vi "UHR-Fleezers Control (host) - 10.2.vi"() -> ()   [LabVIEW 2009] (continued)
                        tunnel: w7403 -> [_ w7436]
                        tunnel: w7402 -> [_ w7427]
                        tunnel: w7392 -> [_ w7434]
                        tunnel: w7401 -> [_ w7433]
                        tunnel: w7390 -> [_ w7432]
                        tunnel: w7400 -> [_ w7431]
                        tunnel: w7385 -> [_ w7429]
                        tunnel: w7384 -> [_ w7428]
                        frame #0 {
                        }
                        frame #1 {
                          n1652 = local read "BD 1 Frequency 3 (MHz)"() -> (w7435:dbl)
                          n1653 = local read "BD 2 Frequency 3 (MHz)"() -> (w7430:dbl)
                          n1654 = local write "Trap Delta (MHz)"(w7427) -> ()
                          n1655 = property on="Initial delta (MHz)" class="DigNum (strict)"("Val(Sgnl)"=w7427) -> ()  [unwired: 2 in, 2 out]
                          n1656 = call "set RF board frequency - interlace.vi"("Board 2 Frequency Limits"=w7428, "Board 1 Frequency Limits"=w7429, "FPGA VI Reference In"=w7436, "Board 2 Frequency 3 (MHz)"=w7430, "Board 1 Frequency 3 (MHz)"=w7435, "Board 2 Frequency 2 (MHz)"=w7431, "Board 2 Frequency 1 (MHz)"=w7432, "Board 1 Frequency 2 (MHz)"=w7433, "Board 1 Frequency 1  (MHz)"=w7434) -> ()  [unwired: 1 in, 2 out]
                          n1657 = local write "BD 2 Frequency 1 (MHz)"(w7432) -> ()
                          n1658 = local write "BD 1 Frequency 1 (MHz)"(w7434) -> ()
                        }
                      }
                    }
                    frame #1 {
                    }
                  }
                }
                event #1 {
                  n1659 = event-data() -> ("Button"=w7437:u16)  [unwired: 8 out]
                  n1660 = case shown="3" w7437 {
                    tunnel: [FALSE TRUE] -> w7438
                    frame #0 {
                    }
                    frame #1 {
                      n1661 = local write "Manipulating Trap"(FALSE ("Manipulating Trap")) -> ()
                    }
                  }
                }
              }
            }
          }
        }
      }
      event #1 {
        n1662 = event-data() -> ()  [unwired: 6 out]
      }
    }
    n1663 = local read "Stop All"() -> (w7259:bool)
    n1664 = node-c288() -> ()  [unwired: 2 out]
  }
  n1665 = timed-loop "Run Scripts, including: stage motion" {
    tunnel: w42 -> [w7444]
    tunnel: w41 -> [w7445]
    tunnel: [w7445] -> w40
    tunnel: [w7444] -> w39
    timing: w37 -> [_]
    timing-out: [_] -> w36
    tunnel: w22 -> [w7443]
    tunnel: w23 -> [w7442]
    stop <- w7446 stop-if-true
    n1666 = node-c288() -> ()  [unwired: 1 in, 1 out]
    n1667 = event shown="[11] \"Take Force FB Data\nUpper Channel\": Value Change" {
      selector: _ -> [_ _ _ _ _ _ _ _ _ _ _ _ _ _ _ _ _]
      dyn-events: _ -> [_ _ _ _ _ _ _ _ _ _ _ _ _ _ _ _ _]
      timeout: _ -> [_ _ _ _ _ _ _ _ _ _ _ _ _ _ _ _ _]
      tunnel: ["Set Position" "Move to Position" "Move Cap. 1 (DNA Right)" "Move Cap. 2 (ADig Left)" _ "Cal/Data Acq. Spot" "Dump Beads" "Dip for Protein" _ _ "Got ADig bead" "Take Force FB Data\nUpper Channel" "Got DNA bead" "Take Stepping Data" _ "Take Detection Laser\nImage" _] -> _
      tunnel: [_ _ _ _ _ _ _ _ _ _ _ _ _ _ _ _ w7961] -> w7446
      tunnel: w7444 -> [w7464 w7472 w7496 w7551 w7596 w7632 w7710 w7735 w7785 w7811 _ w7840 _ _ _ _ _]
      tunnel: w7445 -> [w7465 w7473 w7497 w7552 w7597 w7633 w7711 w7736 w7786 w7812 _ w7841 _ _ _ _ _]
      tunnel: w7443 -> [_ _ w7494 w7548 _ _ _ _ _ _ _ _ _ _ _ _ _]
      tunnel: w7442 -> [_ _ w7493 w7549 _ _ _ _ _ _ _ _ _ _ _ _ _]
      event #0 {
        n1668 = event-data() -> ()  [unwired: 1 in, 5 out]
        n1669 = Build Array("Set Position 1", "Set Position 2", "Set Position 3", "Set Position 4", "Set Position 5") -> (w7463:bool[])
        n1670 = Boolean Array To Number(Boolean array=w7463) -> (number=w7462:u32)
        n1671 = Logarithm Base 2(1:w7462) -> (0:w7454:dbl)
        n1672 = call "Read Stage Position.vi"("error in"=w7464, "VISA resource name in"=w7465) -> ("Current Position"=w7469:cluster{dbl, dbl, dbl}, "error out"=w7468:errorcluster)  [unwired: 2 out]
        n1673 = Decrement(x="Position") -> (x-1=w7452:dbl)
        n1674 = Greater Or Equal?(x=w7454, y=0.0) -> (x >= y?=w7455:bool)
        n1675 = local write "Stage Control Serial Error"(w7468) -> ()
        n1676 = Cluster To Array(cluster=w7469) -> (array=w7466:dbl[])
        n1677 = Select(t=w7454, s=w7455, f=w7452) -> (s? t:f=w7451:dbl)
        n1678 = Increment(x=w7451) -> (x+1=w7450:dbl)
        n1679 = Build Array (concatenate)(w7450, w7466) -> (w7449:dbl[])
        n1680 = Replace Array Subset(array="Saved Stage Positions", new element=w7449, index (row)=w7451) -> (w7467:dbl[][])  [unwired: 1 in]
        n1681 = local write "Saved Stage Positions"(w7467) -> ()
      }
      event #1 {
        n1682 = event-data() -> ()  [unwired: 1 in, 5 out]
        n1683 = flat-sequence {
          tunnel: w7473 -> [w7476]
          tunnel: w7472 -> [w7475]
          frame #0 {
            n1684 = local read "Position"() -> (w7488:dbl)
            n1685 = local read "Saved Stage Positions"() -> (w7486:dbl[][])
            n1686 = Decrement(x=w7488) -> (x-1=w7485:dbl)
            n1687 = Array Subset(array=w7486, index (row)=w7485, length (row)=1 ("length"), index (col)=1 ("index"), length (col)=3 ("length")) -> (w7482:dbl[][])
            n1688 = Reshape Array(w7482, 3 ("dimension size")) -> (w7480:dbl[])
            n1689 = Array To Cluster(array=w7480) -> (cluster=w7479:cluster{"[0]":dbl, "[1]":dbl, "[2]":dbl})
            n1690 = call "Set Stage Position.vi"("Position"=w7479, "error in"=w7475, "VISA resource name in"=w7476) -> ("error out"=w7478:errorcluster)  [unwired: 2 out]
            n1691 = local write "Stage Control Serial Error"(w7478) -> ()
            n1692 = local write "Stage Moving"(TRUE ("Stage Moving")) -> ()
          }
          frame #1 {
            n1693 = call <vilib>:"Beep.vi"() -> ()  [unwired: 3 in, 9 out]
            n1694 = local write "Stage Moving"(FALSE ("Stage Moving")) -> ()
          }
        }
      }
      event #2 {
        n1695 = event-data() -> ()  [unwired: 1 in, 5 out]
        n1696 = local write "Move Cap. 1 (DNA Right)"(FALSE ("Move Cap. 1 (DNA Right)")) -> ()
        n1697 = flat-sequence {
          tunnel: w7497 -> [w7505]
          tunnel: w7496 -> [w7504]
          tunnel: w7494 -> [w7503]
          tunnel: w7493 -> [w7502]
          tunnel: [w7501] -> w7492
          tunnel: [w7500] -> w7491
          tunnel: ["Cap 1 Samp Flow ON"] -> w7490
          tunnel: w7492 -> [w7528]
          tunnel: w7491 -> [w7527]
          tunnel: w7490 -> [w7526]
          frame #0 {
            n1698 = local read "Saved Stage Positions"() -> (w7515:dbl[][])
            n1699 = Array Subset(array=w7515, index (row)=0 ("index"), length (row)=1 ("length"), index (col)=1 ("index"), length (col)=3 ("length")) -> (w7512:dbl[][])
            n1700 = Reshape Array(w7512, 3 ("dimension size")) -> (w7510:dbl[])
            n1701 = Array To Cluster(array=w7510) -> (cluster=w7509:cluster{"[0]":dbl, "[1]":dbl, "[2]":dbl})
            n1702 = case shown="True" "Cap 1 Samp Flow ON" {
              tunnel: w7502 -> [w7517 w7523]
              tunnel: w7503 -> [w7518 w7522]
              tunnel: [w7518 w7520] -> w7501
              tunnel: [w7517 w7519] -> w7500
              frame #0 {
              }
              frame #1 {
                # "run flow"
                n1703 = Concatenate Strings("run" ("string"), "\r") -> (w7524:string)
                n1704 = VISA Write(VISA resource name=w7522, write buffer=w7524, error in (no error)=w7523) -> (VISA resource name out=w7520:refnum<visa-resource-name>, error out=w7519:errorcluster)  [unwired: 1 out]
              }
            }
            n1705 = call "Set Stage Position.vi"("Position"=w7509, "error in"=w7504, "VISA resource name in"=w7505) -> ("error out"=w7508:errorcluster)  [unwired: 2 out]
            n1706 = local write "Stage Control Serial Error"(w7508) -> ()
            n1707 = local write "Stage Moving"(TRUE ("Stage Moving")) -> ()
          }
          frame #1 {
            n1708 = local write "Stage Moving"(FALSE ("Stage Moving")) -> ()
            n1709 = case shown="True" w7526 {
              tunnel: w7527 -> [w7533 w7539]
              tunnel: w7528 -> [w7534 w7538]
              tunnel: [w7534 w7536] -> _
              tunnel: [w7533 w7535] -> _
              frame #0 {
              }
              frame #1 {
                n1710 = Concatenate Strings("stop" ("string"), "\r") -> (w7540:string)
                n1711 = VISA Write(VISA resource name=w7538, write buffer=w7540, error in (no error)=w7539) -> (VISA resource name out=w7536:refnum<visa-resource-name>, error out=w7535:errorcluster)  [unwired: 1 out]
              }
            }
            n1712 = case shown="True" TRUE {
              tunnel: "Cap 1 T ON" -> [w7543 w7544]
              frame #0 {
                n1713 = property on="Trap 1 (ON/OFF)" class="Bool (strict)"("Val(Sgnl)"=w7543) -> ()  [unwired: 2 in, 2 out]
              }
              frame #1 {
                n1714 = property on="Trap 2 (ON/OFF)" class="Bool (strict)"("Val(Sgnl)"=w7544) -> ()  [unwired: 2 in, 2 out]
              }
            }
            n1715 = call <vilib>:"Beep.vi"() -> ()  [unwired: 3 in, 9 out]
            n1716 = case shown="True" "Cap 1 Flow ON" {
              frame #0 {
              }
              frame #1 {
                n1717 = property on="Inject Pump 1" class="Bool (strict)"("Val(Sgnl)"=TRUE ("Value (Signaling)")) -> ()  [unwired: 2 in, 2 out]
              }
            }
          }
        }
      }
      event #3 {
        n1718 = event-data() -> ()  [unwired: 1 in, 5 out]
        n1719 = local write "Move Cap. 2 (ADig Left)"(FALSE ("Move Cap. 2 (ADig Left)")) -> ()
        n1720 = flat-sequence {
          tunnel: w7552 -> [w7560]
          tunnel: w7551 -> [w7559]
          tunnel: w7549 -> [w7558]
          tunnel: w7548 -> [w7557]
          tunnel: [w7556] -> w7547
          tunnel: [w7555] -> w7546
          tunnel: ["Cap 2 Samp Flow ON"] -> w7545
          tunnel: w7547 -> [w7583]
          tunnel: w7546 -> [w7582]
          tunnel: w7545 -> [w7581]
          frame #0 {
            n1721 = local read "Saved Stage Positions"() -> (w7570:dbl[][])
            n1722 = case shown="True" "Cap 2 Samp Flow ON" {
              tunnel: w7558 -> [w7572 w7578]
              tunnel: w7557 -> [w7573 w7577]
              tunnel: [w7573 w7575] -> w7556
              tunnel: [w7572 w7574] -> w7555
              frame #0 {
              }
              frame #1 {
                # "run flow"
                n1723 = Concatenate Strings("run" ("string"), "\r") -> (w7579:string)
                n1724 = VISA Write(VISA resource name=w7577, write buffer=w7579, error in (no error)=w7578) -> (VISA resource name out=w7575:refnum<visa-resource-name>, error out=w7574:errorcluster)  [unwired: 1 out]
              }
            }
            n1725 = Array Subset(array=w7570, index (row)=1 ("index"), length (row)=1 ("length"), index (col)=1 ("index"), length (col)=3 ("length")) -> (w7567:dbl[][])
            n1726 = Reshape Array(w7567, 3 ("dimension size")) -> (w7565:dbl[])
            n1727 = Array To Cluster(array=w7565) -> (cluster=w7564:cluster{"[0]":dbl, "[1]":dbl, "[2]":dbl})
            n1728 = call "Set Stage Position.vi"("Position"=w7564, "error in"=w7559, "VISA resource name in"=w7560) -> ("error out"=w7563:errorcluster)  [unwired: 2 out]
            n1729 = local write "Stage Moving"(TRUE ("Stage Moving")) -> ()
            n1730 = local write "Stage Control Serial Error"(w7563) -> ()
          }
          frame #1 {
            n1731 = local write "Stage Moving"(FALSE ("Stage Moving")) -> ()
            n1732 = case shown="True" TRUE {
              tunnel: "Cap 2 T ON" -> [w7594 w7595]
              frame #0 {
                n1733 = property on="Trap 2 (ON/OFF)" class="Bool (strict)"("Val(Sgnl)"=w7594) -> ()  [unwired: 2 in, 2 out]
              }
              frame #1 {
                n1734 = property on="Trap 1 (ON/OFF)" class="Bool (strict)"("Val(Sgnl)"=w7595) -> ()  [unwired: 2 in, 2 out]
              }
            }
            n1735 = call <vilib>:"Beep.vi"() -> ()  [unwired: 3 in, 9 out]
            n1736 = case shown="True" w7581 {
              tunnel: w7583 -> [_ w7589]
              tunnel: w7582 -> [_ w7588]
              frame #0 {
              }
              frame #1 {
                n1737 = Concatenate Strings("stop" ("string"), "\r") -> (w7591:string)
                n1738 = VISA Write(VISA resource name=w7589, write buffer=w7591, error in (no error)=w7588) -> ()  [unwired: 3 out]
              }
            }
            n1739 = case shown="True" "Cap 2 Flow ON" {
              frame #0 {
              }
              frame #1 {
                n1740 = property on="Inject Pump 3" class="Bool (strict)"("Val(Sgnl)"=TRUE ("Value (Signaling)")) -> ()  [unwired: 2 in, 2 out]
              }
            }
          }
        }
      }
      event #4 {
        n1741 = event-data() -> ()  [unwired: 1 in, 5 out]
        n1742 = flat-sequence {
          tunnel: w7596 -> [w7618]
          tunnel: w7597 -> [w7598]
          frame #0 {
            n1743 = call "Read Stage Position.vi"("error in"=w7618, "VISA resource name in"=w7598) -> ("Current Position"=w7603:cluster{dbl, dbl, dbl}, "error out"=w7616:errorcluster, "VISA resource name out"=w7617:refnum<visa-resource-name>)  [unwired: 1 out]
            n1744 = local read "Saved Stage Positions"() -> (w7627:dbl[][])
            n1745 = Divide(x="z nudge increment (um)", y=1000.0) -> (x/y=w7615:dbl)
            n1746 = Boolean To (0,1)(Boolean="+z") -> (0, 1=w7607:i16)
            n1747 = Boolean To (0,1)(Boolean="-z") -> (0, 1=w7608:i16)
            n1748 = Array Subset(array=w7627, index (row)=1 ("index"), length (row)=1 ("length"), index (col)=1 ("index"), length (col)=3 ("length")) -> (w7624:dbl[][])
            n1749 = Multiply(x=w7607, y=w7615) -> (x*y=w7611:dbl)
            n1750 = Multiply(x=w7608, y=w7615) -> (x*y=w7609:dbl)
            n1751 = Unbundle(w7603) -> (w7601:dbl, w7600:dbl, w7604:dbl)
            n1752 = Negate(x=w7609) -> (-x=w7610:dbl)
            n1753 = Reshape Array(w7624, 3 ("dimension size")) -> (w7622:dbl[])
            n1754 = Add(x=w7611, y=w7610) -> (x+y=w7612:dbl)
            n1755 = Array To Cluster(array=w7622) -> ()  [unwired: 1 out]
            n1756 = Add(x=w7612, y=w7604) -> (x+y=w7602:dbl)
            n1757 = Bundle(cluster=w7603, w7601, w7600, w7602) -> (w7599:cluster{dbl, dbl, dbl})
            n1758 = call "Set Stage Position.vi"("Position"=w7599, "error in"=w7616, "VISA resource name in"=w7617) -> ("error out"=w7621:errorcluster)  [unwired: 2 out]
            n1759 = local write "Stage Moving"(TRUE ("Stage Moving")) -> ()
            n1760 = local write "Stage Control Serial Error"(w7621) -> ()
          }
          frame #1 {
            n1761 = local write "Stage Moving"(FALSE ("Stage Moving")) -> ()
            n1762 = call <vilib>:"Beep.vi"() -> ()  [unwired: 3 in, 9 out]
          }
        }
      }
      event #5 {
        n1763 = event-data() -> ()  [unwired: 1 in, 5 out]
        n1764 = flat-sequence {
          tunnel: w7633 -> [w7636]
          tunnel: w7632 -> [w7635]
          tunnel: ["Cal @ (MHz)"] -> w7630
          tunnel: w7630 -> [w7656]
          tunnel: w7630 -> [w7677]
          frame #0 {
            n1765 = local read "Saved Stage Positions"() -> (w7639:dbl[][])
            n1766 = Array Subset(array=w7639, index (row)=2 ("index"), length (row)=1 ("length"), index (col)=1 ("index"), length (col)=3 ("length")) -> (w7642:dbl[][])
            n1767 = Reshape Array(w7642, 3 ("dimension size")) -> (w7644:dbl[])
            n1768 = local write "Stage Moving"(TRUE ("Stage Moving")) -> ()
            n1769 = Array To Cluster(array=w7644) -> (cluster=w7645:cluster{"[0]":dbl, "[1]":dbl, "[2]":dbl})
            n1770 = call "Set Stage Position.vi"("Position"=w7645, "error in"=w7635, "VISA resource name in"=w7636) -> ("error out"=w7646:errorcluster)  [unwired: 2 out]
            n1771 = local write "Stage Control Serial Error"(w7646) -> ()
          }
          frame #1 {
            n1772 = property on="Trap Delta (MHz)" class="DigNum (strict)"("Val(Sgnl)"="Cal @ (MHz)") -> ()  [unwired: 2 in, 2 out]
            n1773 = local write "Stage Moving"(FALSE ("Stage Moving")) -> ()
            n1774 = call <vilib>:"Beep.vi"() -> ()  [unwired: 3 in, 9 out]
          }
          frame #2 {
            n1775 = Wait (ms)(milliseconds to wait=u32 100) -> ()  [unwired: 1 out]
          }
          frame #3 {
            n1776 = property on="Save Calibration" class="Bool (strict)"("Val(Sgnl)"=TRUE ("Value (Signaling)")) -> ()  [unwired: 2 in, 2 out]
          }
          frame #4 {
            n1777 = Wait (ms)(milliseconds to wait=u32 4000) -> ()  [unwired: 1 out]
          }
          frame #5 {
            n1778 = while {
              stop <- w7653 stop-if-true
              n1779 = local read "Saving..."() -> (w7654:bool)
              n1780 = Wait (ms)(milliseconds to wait=u32 100) -> ()  [unwired: 1 out]
              n1781 = Not(x=w7654) -> (.not. x?=w7653:bool)
            }
          }
          frame #6 {
            n1782 = case shown="True" "W/ Offset 1" {
              tunnel: w7656 -> [_ w7658]
              frame #0 {
              }
              frame #1 {
                n1783 = stacked-sequence {
                  tunnel: w7658 -> [_ _ _ _ _ _ _ w7675]
                  frame #0 {
                    n1784 = property on="Trap Delta (MHz)" class="DigNum (strict)"("Val(Sgnl)"="Offset 1 Start (MHz)") -> ()  [unwired: 2 in, 2 out]
                    n1785 = Replace Array Subset(array=u32[] [0] ("Index Values"), new element="Offset 1 Set", index=0) -> (w7659:u32[])
                    n1786 = property on="Saved AOD Raster Scan Parameter Sets" class="Arr (strict)"("Index Values"=w7659) -> ()  [unwired: 2 in, 2 out]
                  }
                  frame #1 {
                    n1787 = Wait (ms)(milliseconds to wait=u32 200) -> ()  [unwired: 1 out]
                  }
                  frame #2 {
                    n1788 = property on="Load parameters" class="Bool (strict)"("Val(Sgnl)"=TRUE ("Value (Signaling)")) -> ()  [unwired: 2 in, 2 out]
                  }
                  frame #3 {
                    n1789 = Wait (ms)(milliseconds to wait=u32 200) -> ()  [unwired: 1 out]
                  }
                  frame #4 {
                    n1790 = property on="Trap Raster Scan" class="Bool (strict)"("Val(Sgnl)"=TRUE ("Value (Signaling)")) -> ()  [unwired: 2 in, 2 out]
                  }
                  frame #5 {
                    n1791 = Wait (ms)(milliseconds to wait=u32 2000) -> ()  [unwired: 1 out]
                  }
                  frame #6 {
                    n1792 = while {
                      stop <- w7672 stop-if-true
                      n1793 = local read "Raster Scanning..."() -> (w7674:bool)
                      n1794 = local read "Saving..."() -> (w7670:bool)
                      n1795 = Wait (ms)(milliseconds to wait=u32 100) -> ()  [unwired: 1 out]
                      n1796 = Not(x=w7670) -> (.not. x?=w7669:bool)
                      n1797 = Not(x=w7674) -> (.not. x?=w7671:bool)
                      n1798 = And(x=w7671, y=w7669) -> (x .and. y?=w7672:bool)
                    }
                  }
                  frame #7 {
                    n1799 = property on="Trap Delta (MHz)" class="DigNum (strict)"("Val(Sgnl)"=w7675) -> ()  [unwired: 2 in, 2 out]
                  }
                }
              }
            }
          }
          frame #7 {
            n1800 = local read "Save ave N"() -> (w7676:dbl)
            n1801 = case shown="True" "W/ Offset 2" {
              tunnel: w7677 -> [_ w7683]
              tunnel: w7676 -> [_ w7682]
              frame #0 {
                n1802 = Multiply(x="Cal read wait (s)", y=u32 1000 ("milliseconds to wait")) -> (x*y=w7680:u32)
                n1803 = Wait (ms)(milliseconds to wait=w7680) -> ()  [unwired: 1 out]
              }
              frame #1 {
                n1804 = stacked-sequence {
                  tunnel: w7683 -> [_ _ _ _ _ _ _ _ _ w7704 _ _]
                  tunnel: w7682 -> [_ _ _ _ _ _ _ _ _ w7702 _ _]
                  frame #0 {
                    n1805 = property on="Save ave N" class="DigNum (strict)"("Val(Sgnl)"=1.0 ("Value (Signaling)")) -> ()  [unwired: 2 in, 2 out]
                  }
                  frame #1 {
                    n1806 = Wait (ms)(milliseconds to wait=u32 500) -> ()  [unwired: 1 out]
                  }
                  frame #2 {
                    n1807 = property on="Trap Delta (MHz)" class="DigNum (strict)"("Val(Sgnl)"="Offset 2 Start (MHz)") -> ()  [unwired: 2 in, 2 out]
                    n1808 = Replace Array Subset(array=u32[] [0] ("Index Values"), new element="Offset 2 Set", index=0) -> (w7688:u32[])
                    n1809 = property on="Saved AOD Raster Scan Parameter Sets" class="Arr (strict)"("Index Values"=w7688) -> ()  [unwired: 2 in, 2 out]
                  }
                  frame #3 {
                    n1810 = Wait (ms)(milliseconds to wait=u32 500) -> ()  [unwired: 1 out]
                  }
                  frame #4 {
                    n1811 = property on="Load parameters" class="Bool (strict)"("Val(Sgnl)"=TRUE ("Value (Signaling)")) -> ()  [unwired: 2 in, 2 out]
                  }
                  frame #5 {
                    n1812 = Wait (ms)(milliseconds to wait=u32 500) -> ()  [unwired: 1 out]
                  }
                  frame #6 {
                    n1813 = property on="Trap Raster Scan" class="Bool (strict)"("Val(Sgnl)"=TRUE ("Value (Signaling)")) -> ()  [unwired: 2 in, 2 out]
                  }
                  frame #7 {
                    n1814 = Wait (ms)(milliseconds to wait=u32 2000) -> ()  [unwired: 1 out]
                  }
                  frame #8 {
                    n1815 = while {
                      stop <- w7697 stop-if-true
                      n1816 = local read "Raster Scanning..."() -> (w7700:bool)
                      n1817 = local read "Saving..."() -> (w7698:bool)
                      n1818 = Wait (ms)(milliseconds to wait=u32 100) -> ()  [unwired: 1 out]
                      n1819 = Not(x=w7698) -> (.not. x?=w7696:bool)
                      n1820 = Not(x=w7700) -> (.not. x?=w7699:bool)
                      n1821 = And(x=w7699, y=w7696) -> (x .and. y?=w7697:bool)
                    }
                  }
                  frame #9 {
                    n1822 = property on="Trap Delta (MHz)" class="DigNum (strict)"("Val(Sgnl)"=w7704) -> ()  [unwired: 2 in, 2 out]
                    n1823 = property on="Saved AOD Raster Scan Parameter Sets" class="Arr (strict)"("Index Values"=u32[] [0]) -> ()  [unwired: 2 in, 2 out]
                    n1824 = property on="Save ave N" class="DigNum (strict)"("Val(Sgnl)"=w7702) -> ()  [unwired: 2 in, 2 out]
                  }
                  frame #10 {
                    n1825 = Wait (ms)(milliseconds to wait=u32 500) -> ()  [unwired: 1 out]
                  }
                  frame #11 {
                    n1826 = property on="Load parameters" class="Bool (strict)"("Val(Sgnl)"=TRUE ("Value (Signaling)")) -> ()  [unwired: 2 in, 2 out]
                  }
                }
              }
            }
          }
          frame #8 {
            n1827 = property on="Read Cal" class="Bool (strict)"("Val(Sgnl)"=TRUE ("Value (Signaling)")) -> ()  [unwired: 2 in, 2 out]
          }
          frame #9 {
            n1828 = Wait (ms)(milliseconds to wait=u32 500) -> ()  [unwired: 1 out]
          }
          frame #10 {
            n1829 = property on="Fish for Tether" class="Bool (strict)"("Val(Sgnl)"=TRUE ("Value (Signaling)")) -> ()  [unwired: 2 in, 2 out]
          }
        }
        n1830 = local write "Cal/Data Acq. Spot"(FALSE ("Cal/Data Acq. Spot")) -> ()
      }
      event #6 {
        n1831 = event-data() -> ()  [unwired: 1 in, 5 out]
        n1832 = flat-sequence {
          tunnel: w7711 -> [w7717]
          tunnel: w7710 -> [w7716]
          frame #0 {
            w7713 = FALSE ("Fl. Triggered...")
            w7714 = TRUE ("Stage Moving")
            n1833 = local read "Saving..."() -> (w7715:bool)
            n1834 = local write "Fl. Triggered..."(w7713) -> ()
            n1835 = local write "Stage Moving"(w7714) -> ()
            n1836 = property on="Green Laser ON/Interlacing" class="Bool (strict)"("Val(Sgnl)"=w7713) -> ()  [unwired: 2 in, 2 out]
            n1837 = property on="Trap Pos. FB ON" class="Bool (strict)"("Val(Sgnl)"=w7713) -> ()  [unwired: 2 in, 2 out]
            n1838 = local write "Tether"(w7713) -> ()
            n1839 = local write "Stop Saving"(w7715) -> ()
            n1840 = property on="Sample Channel Flow" class="Bool (strict)"("Val(Sgnl)"=w7714) -> ()  [unwired: 2 in, 2 out]
          }
          frame #1 {
            n1841 = local read "Saved Stage Positions"() -> (w7718:dbl[][])
            n1842 = Array Subset(array=w7718, index (row)=3 ("index"), length (row)=1 ("length"), index (col)=1 ("index"), length (col)=3 ("length")) -> (w7723:dbl[][])
            n1843 = Reshape Array(w7723, 3 ("dimension size")) -> (w7721:dbl[])
            n1844 = Array To Cluster(array=w7721) -> (cluster=w7720:cluster{"[0]":dbl, "[1]":dbl, "[2]":dbl})
            n1845 = call "Set Stage Position.vi"("Position"=w7720, "error in"=w7716, "VISA resource name in"=w7717) -> ()  [unwired: 3 out]
          }
          frame #2 {
            w7727 = FALSE ("Value (Signaling)")
            n1846 = property on="Trap 1 (ON/OFF)" class="Bool (strict)"("Val(Sgnl)"=w7727) -> ()  [unwired: 2 in, 2 out]
            n1847 = property on="Trap 2 (ON/OFF)" class="Bool (strict)"("Val(Sgnl)"=w7727) -> ()  [unwired: 2 in, 2 out]
            n1848 = call <vilib>:"Beep.vi"() -> ()  [unwired: 3 in, 9 out]
          }
          frame #3 {
            n1849 = property on="Move Cap. 2 (ADig Left)" class="Bool (strict)"("Val(Sgnl)"=TRUE ("Value (Signaling)")) -> ()  [unwired: 2 in, 2 out]
          }
        }
      }
      event #7 {
        n1850 = event-data() -> ()  [unwired: 1 in, 5 out]
        n1851 = flat-sequence {
          tunnel: w7735 -> [w7739]
          tunnel: w7736 -> [w7740]
          tunnel: [w7740] -> w7730
          tunnel: [w7739] -> w7729
          tunnel: [w7743] -> w7733
          tunnel: [w7742] -> w7731
          tunnel: w7730 -> [w7746]
          tunnel: w7729 -> [w7745]
          tunnel: [w7756] -> w7734
          tunnel: w7733 -> [w7756]
          tunnel: [w7755] -> w7732
          tunnel: w7731 -> [w7755]
          tunnel: w7734 -> [w7761]
          tunnel: w7732 -> [w7760]
          frame #0 {
            n1852 = case shown="True" "Move Trap Before?" {
              frame #0 {
              }
              frame #1 {
                n1853 = property on="Trap Delta (MHz)" class="DigNum (strict)"("Val(Sgnl)"="Dip Trap Delta 1 (MHz)") -> ()  [unwired: 2 in, 2 out]
              }
            }
          }
          frame #1 {
            n1854 = local read "Saved Stage Positions"() -> (w7744:dbl[][])
            n1855 = Array Subset(array=w7744, index (row)=4 ("index"), length (row)=1 ("length"), index (col)=1 ("index"), length (col)=3 ("length")) -> (w7751:dbl[][])
            n1856 = Reshape Array(w7751, 3 ("dimension size")) -> (w7749:dbl[])
            n1857 = Array To Cluster(array=w7749) -> (cluster=w7748:cluster{"[0]":dbl, "[1]":dbl, "[2]":dbl})
            n1858 = call "Set Stage Position.vi"("Position"=w7748, "error in"=w7745, "VISA resource name in"=w7746) -> ("error out"=w7742:errorcluster, "VISA resource name out"=w7743:refnum<visa-resource-name>)  [unwired: 1 out]
          }
          frame #2 {
            n1859 = Multiply(x="Duration (s)", y=1000.0) -> (x*y=w7757:dbl)
            n1860 = Wait (ms)(milliseconds to wait=w7757) -> ()  [unwired: 1 out]
          }
          frame #3 {
            n1861 = local read "Saved Stage Positions"() -> (w7762:dbl[][])
            n1862 = Array Subset(array=w7762, index (row)=2 ("index"), length (row)=1 ("length"), index (col)=1 ("index"), length (col)=3 ("length")) -> (w7767:dbl[][])
            n1863 = Reshape Array(w7767, 3 ("dimension size")) -> (w7765:dbl[])
            n1864 = Array To Cluster(array=w7765) -> (cluster=w7764:cluster{"[0]":dbl, "[1]":dbl, "[2]":dbl})
            n1865 = call "Set Stage Position.vi"("Position"=w7764, "error in"=w7760, "VISA resource name in"=w7761) -> ()  [unwired: 3 out]
          }
          frame #4 {
            n1866 = case shown="True" "Move Trap After?" {
              frame #0 {
              }
              frame #1 {
                n1867 = property on="Trap Delta (MHz)" class="DigNum (strict)"("Val(Sgnl)"="Dip Trap Delta 2 (MHz)") -> ()  [unwired: 2 in, 2 out]
              }
            }
          }
          frame #5 {
            n1868 = case shown="True" "Green ON After?" {
              frame #0 {
              }
              frame #1 {
                n1869 = property on="Green Laser ON/Interlacing" class="Bool (strict)"("Val(Sgnl)"=TRUE ("Value (Signaling)")) -> ()  [unwired: 2 in, 2 out]
              }
            }
          }
          frame #6 {
            n1870 = Wait (ms)(milliseconds to wait=u32 500) -> ()  [unwired: 1 out]
          }
          frame #7 {
            n1871 = case shown="True" "Save Data After?" {
              frame #0 {
              }
              frame #1 {
                n1872 = property on="Start Saving" class="Bool (strict)"("Val(Sgnl)"=TRUE ("Value (Signaling)")) -> ()  [unwired: 2 in, 2 out]
              }
            }
          }
        }
      }
      event #8 {
        n1873 = event-data() -> ()  [unwired: 1 in, 5 out]
        n1874 = flat-sequence {
          tunnel: w7786 -> [w7789]
          tunnel: w7785 -> [w7797]
          tunnel: [w7791] -> w7784
          tunnel: [w7790] -> w7783
          tunnel: [w7788] -> w7781
          tunnel: [w7787] -> w7778
          tunnel: w7784 -> [w7804]
          tunnel: w7783 -> [w7803]
          tunnel: [w7801] -> w7782
          tunnel: w7781 -> [w7802]
          tunnel: [w7800] -> w7780
          tunnel: [w7799] -> w7779
          tunnel: w7778 -> [w7799]
          tunnel: w7782 -> [w7808]
          tunnel: w7780 -> [w7807]
          tunnel: w7779 -> [w7806]
          frame #0 {
            n1875 = call "Read Stage Position.vi"("error in"=w7797, "VISA resource name in"=w7789) -> ("Current Position"=w7787:cluster{dbl, dbl, dbl}, "error out"=w7790:errorcluster, "VISA resource name out"=w7788:refnum<visa-resource-name>)  [unwired: 1 out]
            "Current Position" <- w7787
            n1876 = local write "Stage Control Serial Error"(w7790) -> ()
            n1877 = Unbundle(w7787) -> (w7794:dbl, w7796:dbl, w7792:dbl)
            n1878 = Add(x=w7796, y="Y change (mm)") -> (x+y=w7793:dbl)
            n1879 = Bundle(w7794, w7793, w7792) -> (w7791:cluster{dbl, dbl, dbl})  [unwired: 1 in]
          }
          frame #1 {
            # "move to new position and start saving"
            n1880 = local write "Stage Moving"(TRUE ("Stage Moving")) -> ()
            n1881 = local write "Start Saving"(TRUE ("Start Saving")) -> ()
            n1882 = call "Set Stage Position.vi"("Position"=w7804, "error in"=w7803, "VISA resource name in"=w7802) -> ("error out"=w7800:errorcluster, "VISA resource name out"=w7801:refnum<visa-resource-name>)  [unwired: 1 out]
          }
          frame #2 {
            # "go back to start"
            n1883 = call "Set Stage Position.vi"("Position"=w7806, "error in"=w7807, "VISA resource name in"=w7808) -> ()  [unwired: 3 out]
          }
          frame #3 {
            # "stop saving"
            n1884 = local write "Stop Saving"(TRUE ("Stop Saving")) -> ()
            n1885 = local write "Stage Moving"(FALSE ("Stage Moving")) -> ()
          }
        }
      }
      event #9 {
        n1886 = event-data() -> ()  [unwired: 1 in, 5 out]
        n1887 = Or(x="Move to Position 5", y="Lower Ch. Cap.") -> (x .or. y?=w7814:bool)
        n1888 = Build Array("Move to Position 1", "Move to Position 2", "Move to Position 3", "Move to Position 4", w7814) -> (w7817:bool[])
        n1889 = Boolean Array To Number(Boolean array=w7817) -> (number=w7816:u32)
        n1890 = Logarithm Base 2(1:w7816) -> (0:w7815:dbl)
        n1891 = flat-sequence {
          tunnel: w7815 -> [w7826]
          tunnel: w7812 -> [w7824]
          tunnel: w7811 -> [w7823]
          frame #0 {
            n1892 = local read "Saved Stage Positions"() -> (w7834:dbl[][])
            n1893 = Array Subset(array=w7834, index (row)=w7826, length (row)=1 ("length"), index (col)=1 ("index"), length (col)=3 ("length")) -> (w7831:dbl[][])
            n1894 = Reshape Array(w7831, 3 ("dimension size")) -> (w7829:dbl[])
            n1895 = Array To Cluster(array=w7829) -> (cluster=w7828:cluster{"[0]":dbl, "[1]":dbl, "[2]":dbl})
            n1896 = call "Set Stage Position.vi"("Position"=w7828, "error in"=w7823, "VISA resource name in"=w7824) -> ("error out"=w7827:errorcluster)  [unwired: 2 out]
            n1897 = local write "Stage Moving"(TRUE ("Stage Moving")) -> ()
            n1898 = local write "Stage Control Serial Error"(w7827) -> ()
          }
          frame #1 {
            n1899 = call <vilib>:"Beep.vi"() -> ()  [unwired: 3 in, 9 out]
            n1900 = local write "Stage Moving"(FALSE ("Stage Moving")) -> ()
          }
        }
      }
      event #10 {
        n1901 = event-data() -> ()  [unwired: 1 in, 5 out]
        n1902 = property on="Move Cap. 1 (DNA Right)" class="Bool (strict)"("Val(Sgnl)"=TRUE ("Value (Signaling)")) -> ()  [unwired: 2 in, 2 out]
        n1903 = property on="Inject Pump 3" class="Bool (strict)"("Val(Sgnl)"=FALSE ("Value (Signaling)")) -> ()  [unwired: 2 in, 2 out]
      }
      event #11 {
        n1904 = event-data() -> ()  [unwired: 1 in, 5 out]
        n1905 = flat-sequence {
          tunnel: w7841 -> [w7845]
          tunnel: w7840 -> [w7844]
          frame #0 {
            n1906 = local read "Saved Stage Positions"() -> (w7848:dbl[][])
            n1907 = local write "Stage Moving"(TRUE ("Stage Moving")) -> ()
            n1908 = Array Subset(array=w7848, index (row)=4 ("index"), length (row)=1 ("length"), index (col)=1 ("index"), length (col)=3 ("length")) -> (w7853:dbl[][])
            n1909 = Reshape Array(w7853, 3 ("dimension size")) -> (w7851:dbl[])
            n1910 = Array To Cluster(array=w7851) -> (cluster=w7846:cluster{"[0]":dbl, "[1]":dbl, "[2]":dbl})
            n1911 = call "Set Stage Position.vi"("Position"=w7846, "error in"=w7844, "VISA resource name in"=w7845) -> ("error out"=w7843:errorcluster)  [unwired: 2 out]
            n1912 = local write "Stage Control Serial Error"(w7843) -> ()
          }
          frame #1 {
            n1913 = call <vilib>:"Beep.vi"() -> ()  [unwired: 3 in, 9 out]
            n1914 = property on="Trap Delta (MHz)" class="DigNum (strict)"("Val(Sgnl)"="Starting \nTrap Delta (MHz)") -> ()  [unwired: 2 in, 2 out]
            n1915 = local write "Stage Moving"(FALSE ("Stage Moving")) -> ()
            n1916 = Wait (ms)(milliseconds to wait=u32 1000) -> ()  [unwired: 1 out]
          }
          frame #2 {
            n1917 = property on="Set SP to Reading" class="Bool (strict)"("Val(Sgnl)"=TRUE ("Value (Signaling)")) -> ()  [unwired: 2 in, 2 out]
            n1918 = Wait (ms)(milliseconds to wait=u32 500) -> ()  [unwired: 1 out]
          }
          frame #3 {
            w7862 = TRUE ("Value (Signaling)")
            n1919 = property on="Trap Pos. FB ON" class="Bool (strict)"("Val(Sgnl)"=w7862) -> ()  [unwired: 2 in, 2 out]
            n1920 = property on="Green Laser ON/Interlacing" class="Bool (strict)"("Val(Sgnl)"=w7862) -> ()  [unwired: 2 in, 2 out]
            n1921 = Wait (ms)(milliseconds to wait=u32 500) -> ()  [unwired: 1 out]
          }
          frame #4 {
            n1922 = property on="Start Saving" class="Bool (strict)"("Val(Sgnl)"=TRUE ("Value (Signaling)")) -> ()  [unwired: 2 in, 2 out]
          }
        }
      }
      event #12 {
        n1923 = event-data() -> ()  [unwired: 1 in, 5 out]
        n1924 = property on="Cal/Data Acq. Spot" class="Bool (strict)"("Val(Sgnl)"=TRUE ("Value (Signaling)")) -> ()  [unwired: 2 in, 2 out]
        n1925 = property on="Inject Pump 1" class="Bool (strict)"("Val(Sgnl)"=FALSE ("Value (Signaling)")) -> ()  [unwired: 2 in, 2 out]
      }
      event #13 {
        n1926 = event-data() -> ()  [unwired: 1 in, 5 out]
        n1927 = local read "Save ave N"() -> (w7875:dbl)
        n1928 = flat-sequence {
          tunnel: w7875 -> [w7877]
          tunnel: [w7877] -> w7870
          tunnel: [w7879] -> w7871
          tunnel: w7870 -> [w7879]
          tunnel: [w7881] -> w7872
          tunnel: w7871 -> [w7881]
          tunnel: [w7884] -> w7873
          tunnel: w7872 -> [w7884]
          tunnel: [w7886] -> w7874
          tunnel: w7873 -> [w7886]
          tunnel: [w7888] -> w7868
          tunnel: w7874 -> [w7888]
          tunnel: w7868 -> [w7891]
          tunnel: [w7891] -> w7867
          tunnel: w7867 -> [w7892]
          tunnel: [w7892] -> w7869
          tunnel: w7869 -> [w7898]
          frame #0 {
            n1929 = property on="Save ave N" class="DigNum (strict)"("Val(Sgnl)"="Save ave factor") -> ()  [unwired: 2 in, 2 out]
          }
          frame #1 {
            n1930 = Wait (ms)(milliseconds to wait=u32 100) -> ()  [unwired: 1 out]
          }
          frame #2 {
            n1931 = local read "Offset 2 Start (MHz)"() -> (w7883:dbl)
            n1932 = property on="Saved AOD Raster Scan Parameter Sets" class="Arr (strict)"("Index Values"=u32[] [2]) -> ()  [unwired: 2 in, 2 out]
            n1933 = property on="Trap Delta (MHz)" class="DigNum (strict)"("Val(Sgnl)"=w7883) -> ()  [unwired: 2 in, 2 out]
          }
          frame #3 {
            n1934 = property on="Load parameters" class="Bool (strict)"("Val(Sgnl)"=TRUE ("Value (Signaling)")) -> ()  [unwired: 2 in, 2 out]
          }
          frame #4 {
            n1935 = Wait (ms)(milliseconds to wait=u32 100) -> ()  [unwired: 1 out]
          }
          frame #5 {
            n1936 = property on="Trap Raster Scan" class="Bool (strict)"("Val(Sgnl)"=TRUE ("Value (Signaling)")) -> ()  [unwired: 2 in, 2 out]
          }
          frame #6 {
            n1937 = Wait (ms)(milliseconds to wait=u32 1000) -> ()  [unwired: 1 out]
          }
          frame #7 {
            n1938 = while {
              stop <- w7895 stop-if-true
              n1939 = local read "Raster Scanning..."() -> (w7897:bool)
              n1940 = local read "Saving..."() -> (w7896:bool)
              n1941 = Not(x=w7896) -> (.not. x?=w7893:bool)
              n1942 = Not(x=w7897) -> (.not. x?=w7894:bool)
              n1943 = And(x=w7894, y=w7893) -> (x .and. y?=w7895:bool)
            }
          }
          frame #8 {
            n1944 = property on="Save ave N" class="DigNum (strict)"("Val(Sgnl)"=w7898) -> ()  [unwired: 2 in, 2 out]
          }
        }
      }
      event #14 {
        n1945 = event-data() -> ()  [unwired: 1 in, 5 out]
        n1946 = flat-sequence {
          frame #0 {
            n1947 = property on="Saved AOD Raster Scan Parameter Sets" class="Arr (strict)"("Index Values"=u32[] [1]) -> ()  [unwired: 2 in, 2 out]
          }
          frame #1 {
            n1948 = Multiply(x="N Steps", y="Step Size (nm)") -> (x*y=w7900:dbl)
            n1949 = property on="Scan Speed AOD (nm/s) 2" class="DigNum (strict)"("Value"="Step Size (nm)") -> ()  [unwired: 2 in, 2 out]
            n1950 = property on="Step Size AOD (nm) 2" class="DigNum (strict)"("Value"="Step Size (nm)") -> ()  [unwired: 2 in, 2 out]
            n1951 = property on="Scan Range AOD (nm) 2" class="DigNum (strict)"("Value"=w7900) -> ()  [unwired: 2 in, 2 out]
          }
        }
      }
      event #15 {
        n1952 = event-data() -> ()  [unwired: 1 in, 5 out]
        n1953 = flat-sequence {
          tunnel: [w7928] -> w7918
          tunnel: [w7927] -> w7911
          tunnel: [w7926] -> w7903
          tunnel: [w7931] -> w7919
          tunnel: w7918 -> [w7931]
          tunnel: [w7930] -> w7912
          tunnel: w7911 -> [w7930]
          tunnel: [w7929] -> w7904
          tunnel: w7903 -> [w7929]
          tunnel: [w7935] -> w7920
          tunnel: w7919 -> [w7935]
          tunnel: [w7934] -> w7913
          tunnel: w7912 -> [w7934]
          tunnel: [w7933] -> w7905
          tunnel: w7904 -> [w7933]
          tunnel: [w7941] -> w7921
          tunnel: w7920 -> [w7941]
          tunnel: [w7940] -> w7914
          tunnel: w7913 -> [w7940]
          tunnel: [w7939] -> w7906
          tunnel: w7905 -> [w7939]
          tunnel: [w7945] -> w7922
          tunnel: w7921 -> [w7945]
          tunnel: [w7944] -> w7915
          tunnel: w7914 -> [w7944]
          tunnel: [w7943] -> w7907
          tunnel: w7906 -> [w7943]
          tunnel: [w7949] -> w7923
          tunnel: w7922 -> [w7949]
          tunnel: [w7948] -> w7916
          tunnel: w7915 -> [w7948]
          tunnel: [w7947] -> w7908
          tunnel: w7907 -> [w7947]
          tunnel: [w7953] -> w7924
          tunnel: w7923 -> [w7953]
          tunnel: [w7952] -> w7917
          tunnel: w7916 -> [w7952]
          tunnel: [w7951] -> w7909
          tunnel: w7908 -> [w7951]
          tunnel: w7924 -> [w7959]
          tunnel: w7917 -> [w7958]
          tunnel: [w7956] -> w7910
          tunnel: w7909 -> [w7956]
          tunnel: w7910 -> [w7960]
          frame #0 {
            n1954 = local read "Green Laser ON/Interlacing"() -> (w7928:bool)
            n1955 = local read "Green laser mode"() -> (w7927:enum32{"Laser ON", "Laser OFF", "Interlace"})
            n1956 = local read "Green FB On/Off"() -> (w7926:bool)
          }
          frame #1 {
            n1957 = property on="Green FB On/Off" class="Bool (strict)"("Val(Sgnl)"=FALSE ("Value (Signaling)")) -> ()  [unwired: 2 in, 2 out]
          }
          frame #2 {
            n1958 = property on="Green Laser ON/Interlacing" class="Bool (strict)"("Val(Sgnl)"=TRUE ("Value (Signaling)")) -> ()  [unwired: 2 in, 2 out]
            n1959 = property on="Flip Green Filter" class="Bool (strict)"("Val(Sgnl)"=TRUE ("Value (Signaling)")) -> ()  [unwired: 2 in, 2 out]
            n1960 = property on="Green laser mode" class="RadioBtnsControl (strict)"("Val(Sgnl)"=enum32{"Laser ON", "Laser OFF", "Interlace"}."Laser ON" ("Value (Signaling)")) -> ()  [unwired: 2 in, 2 out]
          }
          frame #3 {
            n1961 = Wait (ms)(milliseconds to wait=u32 500) -> ()  [unwired: 1 out]
          }
          frame #4 {
            n1962 = property on="Confocal Image" class="Bool (strict)"("Val(Sgnl)"=TRUE ("Value (Signaling)")) -> ()  [unwired: 2 in, 2 out]
          }
          frame #5 {
            n1963 = Wait (ms)(milliseconds to wait=u32 2000) -> ()  [unwired: 1 out]
          }
          frame #6 {
            n1964 = while {
              stop <- w7954 stop-if-true
              n1965 = local read "Saving..."() -> (w7955:bool)
              n1966 = Not(x=w7955) -> (.not. x?=w7954:bool)
            }
          }
          frame #7 {
            n1967 = property on="Flip Green Filter" class="Bool (strict)"("Val(Sgnl)"=TRUE ("Value (Signaling)")) -> ()  [unwired: 2 in, 2 out]
            n1968 = property on="Green Laser ON/Interlacing" class="Bool (strict)"("Val(Sgnl)"=w7959) -> ()  [unwired: 2 in, 2 out]
            n1969 = property on="Green laser mode" class="RadioBtnsControl (strict)"("Val(Sgnl)"=w7958) -> ()  [unwired: 2 in, 2 out]
          }
          frame #8 {
            n1970 = property on="Green FB On/Off" class="Bool (strict)"("Val(Sgnl)"=w7960) -> ()  [unwired: 2 in, 2 out]
          }
        }
      }
      event #16 {
        n1971 = event-data() -> ()  [unwired: 1 in, 5 out]
        n1972 = local read "Stop All"() -> (w7961:bool)
      }
    }
    n1973 = node-c288() -> ()  [unwired: 1 in, 1 out]
  }
  n1974 = flat-sequence "Video" {
    tunnel: [w7970] -> w38
    tunnel: w38 -> [w8011]
    frame #0 {
      n1975 = while {
        stop <- w7963 continue-if-true
        n1976 = call "Close Video Capture.vi"() -> ("error code OUT"=w7965:i32)
        n1977 = Equal?(x=w7965, y=0) -> (x = y?=w7963:bool)
      }
      n1978 = local write "Stop All"(FALSE ("Stop All")) -> ()
    }
    frame #1 {
      n1979 = call "DMR_Init.vi"() -> ()  [unwired: 3 out]
    }
    frame #2 {
      # "Setting the destination format to Mono8 makes sure that the image can be displayed in the intensity plot."
      n1980 = call "DMR_GetDevice.vi"("search string IN"="DE019116701") -> ("device handle OUT"=w7988:i32)  [unwired: 4 in, 2 out]
      n1981 = call "DMR_OpenDevice.vi"("device handle IN"=w7988) -> ("driver handle OUT"=w7971:i32)  [unwired: 4 out]
      n1982 = call "DMR_FindList.vi"("flags IN"=u32 0 ("flags"), "list name IN"="" ("String"), "list type IN"=T47."camera descriptions", "driver handle IN"=w7971) -> ("list handle OUT"=w7974:i32)  [unwired: 2 out]
      n1983 = call "DMR_FindList.vi"("flags IN"=u32 0 ("flags"), "list name IN"="Base", "list type IN"=T47."setting", "driver handle IN"=w7971) -> ("list handle OUT"=w7972:i32)  [unwired: 2 out]
      n1984 = call "OBJ_GetHandle.vi"("object name IN"="VideoStandard", "list handle IN"=w7974) -> ("object handle OUT"=w7968:i32)  [unwired: 3 out]
      n1985 = call "OBJ_GetHandle.vi"("object name IN"="PixelFormat", "list handle IN"=w7972) -> ("object handle OUT"=w7982:i32)  [unwired: 3 out]
      n1986 = call "OBJ_SetS.vi"("value index IN"=0, "value IN"="NTSC M", "object handle IN"=w7968) -> ()  [unwired: 2 out]
      n1987 = call "OBJ_SetS.vi"("value index IN"=0, "value IN"="Mono8" ("value"), "object handle IN"=w7982) -> ()  [unwired: 2 out]
      n1988 = call "OBJ_GetHandle.vi"("object name IN"="VideoChannel", "list handle IN"=w7972) -> ("object handle OUT"=w7978:i32)  [unwired: 3 out]
      n1989 = while {
        tunnel: [w7993] -> w7970
        tunnel: w7971 -> [w7990]
        stop <- w7991 continue-if-true
        n1990 = call "DMR_ImageRequestSingle.vi"("request control IN"=0, "driver handle IN"=w7990) -> ("error code OUT"=w7992:i32, "driver handle OUT"=w7993:i32)  [unwired: 2 out]
        n1991 = Equal To 0?(x=w7992) -> (x = 0?=w7991:bool)
      }
      n1992 = call "OBJ_SetI.vi"("value index IN"=0, "value IN"=3 ("Video channel"), "object handle IN"=w7978) -> ()  [unwired: 2 out]
    }
    frame #3 {
      w7999 = T17 0 items=["Grayscale (U8)", "Grayscale (I16)", "Grayscale (SGL)", "Complex (CSG)", "RGB (U32)", "HSL (U32)", "RGB (U64)"] ("Image Type")
      w8007 = T17 0 items=["Grayscale (U8)", "Grayscale (I16)", "Grayscale (SGL)", "Complex (CSG)", "RGB (U32)", "HSL (U32)", "RGB (U64)"] ("Image Type")
      n1993 = for "Create Greyscale map" {
        N: 256 -> [_]
        tunnel: [w8013] -> w7996 mode=indexing
        workers-P: _ -> [_]
        i -> [w8016]
        n1994 = To Unsigned Byte Integer(number=w8016) -> (unsigned 8bit integer=w8012:u8)
        n1995 = Join Numbers(hi=w8012, lo=w8012) -> ((hi.lo)=w8015:u16)
        n1996 = Join Numbers(hi=w8012, lo=w8012) -> ((hi.lo)=w8014:u16)
        n1997 = Join Numbers(hi=w8015, lo=w8014) -> ((hi.lo)=w8013:u32)
      }
      n1998 = call "IMAQ Create"("Image Name"="Scaled video", "Image Type"=w7999) -> ("New Image"=w7998:T2)  [unwired: 2 in, 2 out]
      n1999 = call "IMAQ Create"("Image Name"="Main video", "Image Type"=w8007) -> ("New Image"=w8008:T2)  [unwired: 2 in, 2 out]
      n2000 = node-c288(0 ("Processor")) -> (w8006:T23)  [unwired: 3 out]
      n2001 = Initialize Array(u32 0 ("Window Number (0...15)"), 480 ("dimension size"), 640 ("dimension size")) -> (w8001:u32[][])
      n2002 = timed-loop {
        tunnel: w8011 -> [w8033]
        tunnel: [w8032] -> w8010
        tunnel: w8008 -> [w8031]
        timing: w8006 -> [_]
        timing-out: [_] -> w8005
        tunnel: w8001 -> [w8020]
        tunnel: w7998 -> [w8018]
        tunnel: w7996 -> [w8017]
        stop <- w8019 stop-if-true
        # "This block performs the \nactual image capture."
        n2003 = node-c288() -> ()  [unwired: 2 out]
        n2004 = local read "Stop All"() -> (w8019:bool)
        n2005 = Reciprocal(x="Video Capture Rate (Hz)") -> (1/x=w8023:dbl)
        n2006 = Multiply(x=w8023, y=1000.0) -> (x*y=w8021:dbl)
        n2007 = call "DMR_ImageRequestWaitFor.vi"("queue number IN"=0, "timeout(ms) IN"=500, "driver handle IN"=w8033) -> ("error code OUT"=w8037:i32, "request number OUT"=w8034:i32, "driver handle OUT"=w8035:i32)
        n2008 = feedback #31(T48 refnum ("Avi Refnum")) -> (w8025:T48)
        n2009 = case shown="True" "New Video File" {
          tunnel: [T48 refnum ("Avi Refnum") w8054] -> w8027
          tunnel: [FALSE TRUE] -> w8028
          tunnel: w8025 -> [_ w8050]
          frame #0 {
          }
          frame #1 {
            n2010 = call "Create new save file.vi"("Ext"=".avi" ("string"), "Index In"="Video Index") -> ("Path Out"=w8046:path, "Index Out"=w8047:dbl)  [unwired: 1 in]
            "Path Out" <- w8046
            n2011 = Not Equal?(x=w8050, y=T48 refnum ("Avi Refnum")) -> (x != y?=w8051:bool)
            n2012 = Increment(x=w8047) -> (x+1=w8056:dbl)
            n2013 = case shown="True" w8051 {
              tunnel: w8050 -> [_ w8057]